vi "HFRR ADV v042.vi"() -> ()   [LabVIEW 2025] (continued)
                n2720 = local read "clk"() -> (w3226:dbl)
                n2721 = Equal?(x=w3226, y=10.0) -> (x = y?=w3228:bool)
                n2722 = case shown="True" w3233 {
                  tunnel: w3232 -> [_ w3359]
                  tunnel: [FALSE ("Boolean 2") TRUE ("Boolean 2")] -> _
                  frame False {
                  }
                  frame True {
                    w3313 = ";" ("Substring")
                    # "Pid out/\nFreq response value"
                    n2723 = local write "act save time"(w3359) -> ()
                    n2724 = local read "FILE"() -> (w3307:string)
                    n2725 = call "file check.vi"("file name in"=w3307) -> ("error out"=w3310:errorcluster, "file name out"=w3305:string)  [unwired: 9 in]
                    n2726 = local read "LVDT STROKE"() -> (w3302:dbl)
                    n2727 = local read "Add up Stroke"() -> (w3300:dbl)
                    n2728 = call "FILE PATH CREATION.vi"("error in"=w3310, "FILE NAME :"=w3305) -> ("FILE OUT"=w3308:path)  [unwired: 8 in, 1 out]
                    n2729 = local read "STROKE Initialize"() -> (w3295:bool)
                    n2730 = Concatenate Strings(w3305, ".dgf" ("Substring")) -> (w3309:string)
                    n2731 = Subtract(x=w3302, y=w3300) -> (x-y=w3301:dbl)
                    n2732 = Absolute Value(x=w3301) -> (abs(x)=w3298:dbl)
                    n2733 = local read "FF 2"() -> (→"Frictional Force ( N )" →"Frictional Force ( N )":dbl)
                    n2734 = Build Path(base path=w3308, name or relative path=w3309) -> (appended path=w3304:path)
                    n2735 = flat-sequence {
                      tunnel: w3298 -> [w3364]
                      tunnel: [w3363] -> w3296
                      tunnel: w3295 -> [w3361]
                      tunnel: [w3366] -> w3297
                      tunnel: w3296 -> [w3366]
                      frame #0 {
                        n2736 = call <vilib>:"Mean PtByPt.vi"("x"=w3364, "sample length"="STROKE FILTER", "initialize"=w3361) -> ("mean"=w3363:dbl)  [unwired: 1 in, 1 out]
                      }
                      frame #1 {
                        "STROKE Initialize" <- FALSE ("STROKE Initialize")
                      }
                    }
                    n2737 = local read "COF 2"() -> (w3318:dbl)
                    "Coefficient of Friction" <- w3318
                    "COF 4" <- w3318
                    "Coefficient of Friction" <- w3318
                    n2738 = local read "TEMP"() -> (w3321:dbl)
                    "Temperature ( Deg C )" <- w3321
                    n2739 = local read "Humidity ( %RH )"() -> (w3320:dbl)
                    n2740 = local read "Frequency ( Hz )"() -> (w3327:dbl)
                    n2741 = local read "LVDT STROKE DISPLAY"() -> (w3299:dbl)
                    n2742 = local read "Elapsed time"() -> (w3352:dbl)
                    n2743 = local read "AIR TEMP"() -> (w3325:dbl)
                    n2744 = local read "PID-out"() -> (w3330:dbl)
                    n2745 = local write "Temperature ( Deg C )"(w3321) -> ()
                    n2746 = Number To Fractional String(number=w3299, width (-)=i16 9 ("precision (6)"), precision (6)=i16 6) -> (F-format string=w3345:string)  [unwired: 1 in]
                    n2747 = Number To Fractional String(number=w3325, width (-)=i16 9 ("precision (6)"), precision (6)=i16 3) -> (F-format string=w3344:string)  [unwired: 1 in]
                    n2748 = Number To Fractional String(number=w3321, width (-)=i16 9 ("precision (6)"), precision (6)=i16 3) -> (F-format string=w3341:string)  [unwired: 1 in]
                    n2749 = Number To Fractional String(number=w3320, width (-)=i16 9 ("precision (6)"), precision (6)=i16 3) -> (F-format string=w3338:string)  [unwired: 1 in]
                    n2750 = Number To Fractional String(number=0.0, width (-)=i16 9 ("precision (6)"), precision (6)=i16 3) -> (F-format string=w3335:string)  [unwired: 1 in]
                    n2751 = Number To Fractional String(number=w3330, width (-)=i16 9 ("precision (6)"), precision (6)=i16 3) -> (F-format string=w3331:string)  [unwired: 1 in]
                    n2752 = Number To Fractional String(number=w3327, width (-)=i16 9 ("precision (6)"), precision (6)=i16 3) -> (F-format string=w3326:string)  [unwired: 1 in]
                    n2753 = Number To Fractional String(number=w3318, width (-)=i16 9 ("precision (6)"), precision (6)=i16 6) -> (F-format string=w3353:string)  [unwired: 1 in]
                    n2754 = Number To Fractional String(number=w3352, width (-)=i16 14 ("precision (6)"), precision (6)=i16 3) -> (F-format string=w3354:string)  [unwired: 1 in]
                    n2755 = Bundle("y"=1.02, "LVDT STROKE DISPLAY"=w3299, "y"=0.98) -> (w3319:T30)  [unwired: 1 in]
                    n2756 = Number To Fractional String(number="Ambient Humidity :", width (-)=i16 9 ("precision (6)"), precision (6)=i16 6) -> (F-format string=w3311:string)  [unwired: 1 in]
                    n2757 = local read "RUN"() -> (w3317:bool)
                    n2758 = case shown="True" w3317 {
                      tunnel: w3319 -> [_ w3370]
                      tunnel: w3299 -> [_ w3369]
                      tunnel: w3299 -> [_ w3367]
                      tunnel: w3299 -> [_ w3368]
                      frame False {
                      }
                      frame True {
                        "Stroke ( mm )" <- w3370
                        "Stroke ( mm )" <- w3370
                        "Stroke 4" <- w3369
                        "Stroke 3" <- w3367
                        "Stroke 2" <- w3368
                        "measured_stroke" <- w3367
                      }
                    }
                    n2759 = Concatenate Strings(w3354, w3313, w3353, w3313, w3345, w3313, w3344, w3313, w3341, w3313, w3338, w3313, w3335, w3313, w3331, w3313, w3326, w3313, w3311, "\r") -> (w3351:string)
                    n2760 = call <vilib>:"Write Characters To File.vi"("append to file? (new file:F)"=TRUE, "character string"=w3351, "file path (dialog if empty)"=w3304) -> ()  [unwired: 2 in, 1 out]
                    "refresh flag" <- TRUE ("refresh flag")
                    "LVDT STROKE Actual" <- w3297
                  }
                }
                n2761 = case shown="True" w3219 {
                  tunnel: w3229 -> [_ w3255]
                  tunnel: w3234 -> [_ w3265]
                  tunnel: [0.0 w3261] -> _
                  tunnel: w3228 -> [_ w3260]
                  tunnel: [0.0 w3259] -> _
                  tunnel: w3218 -> [_ w3259]
                  tunnel: w3232 -> [w3248 _]
                  frame False {
                    n2762 = local write "acq timer"(w3248) -> ()
                    n2763 = local write "Test Duration Status"(0.0 ("Test Duration Status")) -> ()
                  }
                  frame True {
                    n2764 = local read "Set Hz"() -> (w3262:dbl)
                    n2765 = local write "Elapsed time"(w3255) -> ()
                    n2766 = local read "test time"() -> (w3254:dbl)
                    n2767 = Multiply(x=w3265, y=w3262) -> (x*y=w3264:dbl)
                    n2768 = case shown="False" w3260 {
                      tunnel: w3264 -> [w3266 _]
                      tunnel: [w3266 1.0] -> w3261
                      frame False {
                        n2769 = local write "Cycles elapsed"(w3266) -> ()
                      }
                      frame True {
                      }
                    }
                    n2770 = Greater?(x=w3255, y=w3254) -> (0:w3263:bool)
                    n2771 = Subtract(x=w3254, y=w3255) -> (x-y=w3253:dbl)
                    n2772 = Multiply(x=w3253, y=60.0) -> (x*y=w3252:dbl)
                    n2773 = local write "Time Remaining"(w3252) -> ()
                    n2774 = local write "Remaining Time"(w3252) -> ()
                    n2775 = case shown="True" w3263 {
                      frame False {
                      }
                      frame True {
                        n2776 = stacked-sequence {
                          frame #0 {
                            w3271 = T19."Enabled" ("Disabled")
                            w3270 = FALSE ("TEST FILE NAM,E SAVED")
                            w3272 = "" ("FILE")
                            w3273 = TRUE ("Visible")
                            n2777 = local write "Humidity"(FALSE ("Humidity")) -> ()
                            n2778 = local write "RUN"(FALSE ("OK Button 2")) -> ()
                            n2779 = local write "Heater Button"(FALSE ("Heater Button")) -> ()
                            n2780 = local write "Auto Start Test"(FALSE ("Auto Start Test")) -> ()
                            n2781 = local write "TestCompFlg"(TRUE ("StpFlg")) -> ()
                            n2782 = local read "Humidity ( %RH )"() -> (→"Rh After":dbl)
                            n2783 = property on="STOP 2" class="Bool (strict)"("Disabled"=u8 0) -> ()  [unwired: 2 in, 2 out]
                            n2784 = local read "EVENT LOG"() -> (w3278:string)
                            n2785 = call "Event Log.vi"("Content"="Test Completed", "EVENT LOG"=w3278) -> ("EVENT LOG"=w3277:string)  [unwired: 8 in, 1 out]
                            n2786 = property on="RUN" class="Bool (strict)"("Visible"=w3273) -> ()  [unwired: 2 in, 2 out]
                            n2787 = property on="Auto Start Test" class="Bool (strict)"("Visible"=w3273) -> ()  [unwired: 2 in, 2 out]
                            n2788 = local write "Batch Ref Num :"(w3272) -> ()
                            n2789 = local write "FILE"(w3272) -> ()
                            n2790 = local write "EVENT LOG"(w3277) -> ()
                            n2791 = local write "TEST FILE NAM,E SAVED"(w3270) -> ()
                            n2792 = local write "Fuel Discription :"(w3272) -> ()
                            n2793 = local write "START TEMP"(w3270) -> ()
                            n2794 = local write "Remarks :"(w3272) -> ()
                            n2795 = local write "Main Dashboard Buttons"(T1."Imaging" ("Main Dashboard Buttons")) -> ()
                            n2796 = local write "Main Tab"(T2."Adv Scar" ("Main Tab")) -> ()
                            n2797 = property on="FRICVALZ 2" class="Bool (strict)"("DisabledEnum"=w3271) -> ()  [unwired: 2 in, 2 out]
                            n2798 = property on="FRICVALZ 3" class="Bool (strict)"("DisabledEnum"=w3271) -> ()  [unwired: 2 in, 2 out]
                            n2799 = property on="FRICVALZ 4" class="Bool (strict)"("DisabledEnum"=w3271) -> ()  [unwired: 2 in, 2 out]
                          }
                          frame #1 {
                            n2800 = Wait (ms)(milliseconds to wait=u32 1500) -> ()  [unwired: 1 out]
                          }
                          frame #2 {
                            n2801 = local write "Due Write"("VC;0") -> ()
                          }
                          frame #3 {
                            n2802 = Wait (ms)(milliseconds to wait=u32 1500) -> ()  [unwired: 1 out]
                          }
                          frame #4 {
                            n2803 = local write "Due Write"("VC;0") -> ()
                          }
                          frame #5 {
                            n2804 = Wait (ms)(milliseconds to wait=u32 1500) -> ()  [unwired: 1 out]
                          }
                          frame #6 {
                            n2805 = local write "Due Write"("ST;0") -> ()
                          }
                          frame #7 {
                            n2806 = local write "measured_stroke"(0.0 ("measured_stroke")) -> ()
                            n2807 = Wait (ms)(milliseconds to wait=u32 1500) -> ()  [unwired: 1 out]
                          }
                          frame #8 {
                            n2808 = local write "Due Write"("HE;0") -> ()
                            n2809 = local write "Humidity 2"(TRUE ("Humidity")) -> ()
                          }
                        }
                      }
                    }
                    n2810 = Divide(x=w3255, y=w3254) -> (x/y=w3258:dbl)
                    n2811 = Multiply(x=w3258, y=100.0) -> (x*y=w3256:dbl)
                    n2812 = local write "Test Duration Status"(w3256) -> ()
                  }
                }
              }
              frame #2 {
                n2813 = case shown="True" "Heater Button" {
                  tunnel: [0.0 ("output") w3393] -> w3371
                  frame False {
                    w3374 = TRUE ("tmpchk")
                    n2814 = local read "TEMP"() -> (w3375:dbl)
                    n2815 = local write "Temp ini"(w3375) -> ()
                    n2816 = local write "Reset 4"(w3374) -> ()
                    n2817 = local write "tmpchk"(w3374) -> ()
                    n2818 = local write "reinit"(TRUE ("reinit")) -> ()
                    n2819 = local write "manual temp log"(TRUE ("manual temp log")) -> ()
                  }
                  frame True {
                    # "Logic to turn off\nthe heater when \ntemp is not rising.\nTime - 60 sec\nDelta t- 5°c"
                    n2820 = local read "Temp ini"() -> (w3382:dbl)
                    n2821 = local read "Auto Start Test"() -> (w3378:bool)
                    n2822 = Less?(x=w3382, y=53.0) -> (x < y?=w3380:bool)
                    n2823 = case shown="False" w3378 {
                      frame False {
                        n2824 = local read "Set Temp"() -> (w3402:dbl)
                        n2825 = local read "TEMP"() -> (w3401:dbl)
                        n2826 = Subtract(x=w3402, y=w3401) -> (x-y=w3400:dbl)
                        n2827 = Absolute Value(x=w3400) -> (abs(x)=w3399:dbl)
                        n2828 = Less?(x=w3399, y=0.5) -> (x < y?=w3397:bool)
                        n2829 = case shown="True" w3397 {
                          tunnel: "manual temp log" -> [_ w3403]
                          frame False {
                          }
                          frame True {
                            n2830 = case shown="True" w3403 {
                              selector: w3403 -> [_ w3404]
                              frame False {
                              }
                              frame True {
                                # "#Event log"
                                n2831 = Not(x=w3404) -> (.not. x?=w3405:bool)
                                n2832 = local write "manual temp log"(w3405) -> ()
                                n2833 = local read "EVENT LOG"() -> (w3408:string)
                                n2834 = call "Event Log.vi"("Content"="Target Temperature reached", "EVENT LOG"=w3408) -> ("EVENT LOG"=w3407:string)  [unwired: 8 in, 1 out]
                                n2835 = local write "EVENT LOG"(w3407) -> ()
                              }
                            }
                          }
                        }
                      }
                      frame True {
                        n2836 = local write "manual temp log"(TRUE ("manual temp log")) -> ()
                      }
                    }
                    n2837 = And(x="tmpchk", y=w3380) -> (x .and. y?=w3383:bool)
                    n2838 = case shown="True" w3383 {
                      frame False {
                      }
                      frame True {
                        n2839 = call "Elapsed Time8"("Time Target (s)"=300.0, "Reset"="Reset 4") -> ("Time has Elapsed"=w3410:bool)  [unwired: 10 in, 7 out]
                        n2840 = flat-sequence {
                          tunnel: w3410 -> [_]
                          frame #0 {
                            n2841 = local write "Reset 4"(FALSE ("Reset 4")) -> ()
                          }
                        }
                        n2842 = case shown="True" w3410 {
                          frame False {
                          }
                          frame True {
                            n2843 = local read "Temp ini"() -> (w3417:dbl)
                            n2844 = Add(x=w3417, y=5.0) -> (x+y=w3415:dbl)
                            n2845 = local read "TEMP"() -> (w3418:dbl)
                            n2846 = Greater?(x=w3418, y=w3415) -> (0:w3416:bool)
                            n2847 = case shown="False" w3416 {
                              frame False {
                                n2848 = local write "Heater Button"(FALSE ("Heater Button")) -> ()
                              }
                              frame True {
                                n2849 = local write "tmpchk"(FALSE ("tmpchk")) -> ()
                              }
                            }
                          }
                        }
                      }
                    }
                    n2850 = local read "Set Temp"() -> (w3391:dbl)
                    n2851 = local read "TEMP"() -> (w3385:dbl)
                    n2852 = call-poly <vilib>:"PID.vi"("reinitialize? (F)"="reinit", "dt (s)"=-1.0, "process variable"=w3385, "setpoint"=w3391) -> ("output"=w3388:dbl)  [unwired: 6 in, 1 out]
                    n2853 = Subtract(x=w3391, y=w3385) -> (x-y=w3392:dbl)
                    n2854 = Add(x=w3391, y=0.5) -> (x+y=w3389:dbl)
                    n2855 = Greater Or Equal?(x=w3385, y=w3389) -> ()  [unwired: 1 out]
                    n2856 = Select(t=0.0, s=FALSE, f=w3388) -> (s? t:f=w3387:dbl)
                    "PID output" <- w3387
                    n2857 = flat-sequence {
                      tunnel: w3387 -> [w3421]
                      tunnel: [w3421] -> w3393
                      frame #0 {
                        n2858 = local write "reinit"(FALSE ("reinit")) -> ()
                      }
                    }
                    n2859 = Bundle(w3392, "output"=w3387, "TEMP"=w3385) -> ()  [unwired: 1 in, 1 out]
                  }
                }
                "PID-out" <- w3371
              }
              frame #3 {
                n2860 = local read "TEMP"() -> (w3423:dbl)
                n2861 = Greater Or Equal?(x=w3423, y="Set Temp 2") -> (x >= y?=w3428:bool)
                n2862 = case shown="True" w3428 {
                  tunnel: [FALSE TRUE] -> w3426
                  frame False {
                  }
                  frame True {
                  }
                }
                "Status 13" <- w3426
                n2863 = And(x=w3426, y="trip1 8") -> (x .and. y?=w3425:bool)
                n2864 = case shown="True" w3425 {
                  frame False {
                    n2865 = local write "Heater Trip Temp"(TRUE ("Heater Trip Temp")) -> ()
                  }
                  frame True {
                    w3431 = FALSE ("OK Button 2")
                    n2866 = case shown="True" "Heater Trip Temp" {
                      selector: "Heater Trip Temp" -> [_ w3433]
                      frame False {
                      }
                      frame True {
                        n2867 = Not(x=w3433) -> (.not. x?=w3432:bool)
                        n2868 = local read "EVENT LOG"() -> (w3436:string)
                        n2869 = local write "Heater Trip Temp"(w3432) -> ()
                        n2870 = call "Event Log.vi"("Content"="Heater Trip", "EVENT LOG"=w3436) -> ("EVENT LOG"=w3435:string)  [unwired: 8 in, 1 out]
                        n2871 = local write "EVENT LOG"(w3435) -> ()
                      }
                    }
                    n2872 = local write "RUN"(w3431) -> ()
                    n2873 = property on="Auto Start Test" class="Bool (strict)"("Value"=w3431) -> ()  [unwired: 2 in, 2 out]
                    n2874 = local write "Heater Button"(w3431) -> ()
                  }
                }
              }
            }
            n2875 = case shown="False" w3142 {
              frame False {
                n2876 = disable-structure shown="Disabled" {
                  frame Disabled {
                    n2877 = stacked-sequence {
                      frame #0 {
                        n2878 = local write "RUN"(FALSE ("OK Button 2")) -> ()
                      }
                      frame #1 {
                      }
                    }
                  }
                  frame Enabled {
                  }
                }
              }
              frame True {
              }
            }
          }
        }
        n2879 = local read "Reset Graph"() -> (w3039:bool)
        n2880 = case shown="True" w3039 {
          selector: w3039 -> [_ w3056]
          frame False {
          }
          frame True {
            w3070 = 0.0 ("X Scale.Range:Maximum")
            n2881 = Not(x=w3056) -> (.not. x?=w3055:bool)
            n2882 = local write "Reset Graph"(w3055) -> ()
            n2883 = property on="Electrical Contact Resistance ( % )" class="WFChart (strict)"("XScale.Maximum"=600.0 ("X Scale.Range:Maximum"), "XScale.Minimum"=0.0 ("X Scale.Range:Minimum"), "YScale.Maximum"=100.0 ("Y Scale.Range:Maximum"), "YScale.Minimum"=0.0 ("Y Scale.Range:Minimum")) -> ()  [unwired: 2 in, 2 out]
            n2884 = property on="Frictional Force ( N )" class="WFChart (strict)"("XScale.Maximum"=600.0 ("X Scale.Range:Maximum"), "XScale.Minimum"=0.0 ("X Scale.Range:Minimum"), "YScale.Maximum"=100.0 ("Y Scale.Range:Maximum"), "YScale.Minimum"=0.0 ("Y Scale.Range:Minimum")) -> ()  [unwired: 2 in, 2 out]
            n2885 = property on="Temperature ( Deg C )" class="WFChart (strict)"("XScale.Maximum"=600.0 ("X Scale.Range:Maximum"), "XScale.Minimum"=0.0 ("X Scale.Range:Minimum"), "YScale.Maximum"=100.0 ("Y Scale.Range:Maximum"), "YScale.Minimum"=0.0 ("Y Scale.Range:Minimum")) -> ()  [unwired: 2 in, 2 out]
            n2886 = property on="Stroke ( mm )" class="WFChart (strict)"("XScale.Maximum"=600.0 ("X Scale.Range:Maximum"), "XScale.Minimum"=0.0 ("X Scale.Range:Minimum"), "YScale.Maximum"=100.0 ("Y Scale.Range:Maximum"), "YScale.Minimum"=0.0 ("Y Scale.Range:Minimum")) -> ()  [unwired: 2 in, 2 out]
            n2887 = property on="Coefficient of Friction" class="WFChart (strict)"("XScale.Maximum"=600.0 ("X Scale.Range:Maximum"), "XScale.Minimum"=0.0 ("X Scale.Range:Minimum"), "YScale.Maximum"=100.0 ("Y Scale.Range:Maximum"), "YScale.Minimum"=0.0 ("Y Scale.Range:Minimum")) -> ()  [unwired: 2 in, 2 out]
            n2888 = property on="Electrical Contact Resistance ( % )" class="WFChart (strict)"("XScale.Minimum"=0.0 ("X Scale.Range:Minimum"), "XScale.Maximum"=600.0 ("X Scale.Range:Maximum"), "YScale.Minimum"=0.0 ("Y Scale.Range:Minimum"), "YScale.Maximum"=100.0 ("Y Scale.Range:Maximum")) -> ()  [unwired: 2 in, 2 out]
            n2889 = property on="Temperature ( Deg C )" class="WFChart (strict)"("XScale.Minimum"=0.0 ("X Scale.Range:Minimum"), "XScale.Maximum"=600.0 ("X Scale.Range:Maximum"), "YScale.Minimum"=0.0 ("Y Scale.Range:Minimum"), "YScale.Maximum"=100.0 ("Y Scale.Range:Maximum")) -> ()  [unwired: 2 in, 2 out]
            n2890 = property on="Coefficient of Friction" class="WFChart (strict)"("XScale.Minimum"=0.0 ("X Scale.Range:Minimum"), "XScale.Maximum"=600.0 ("X Scale.Range:Maximum"), "YScale.Maximum"=1.0 ("X Scale.Range:Minimum"), "YScale.Minimum"=0.0 ("X Scale.Range:Minimum")) -> ()  [unwired: 2 in, 2 out]
            n2891 = property on="Frictional Force ( N )" class="WFChart (strict)"("XScale.Maximum"=600.0 ("X Scale.Range:Maximum"), "XScale.Minimum"=w3070, "YScale.Maximum"=10.0 ("Y Scale.Range:Maximum"), "YScale.Minimum"=w3070) -> ()  [unwired: 2 in, 2 out]
            n2892 = property on="Stroke ( mm )" class="WFChart (strict)"("XScale.Maximum"=600.0 ("X Scale.Range:Maximum"), "XScale.Minimum"=0.0 ("X Scale.Range:Minimum"), "YScale.Maximum"=100.0 ("Y Scale.Range:Maximum"), "YScale.Minimum"=0.0 ("Y Scale.Range:Minimum")) -> ()  [unwired: 2 in, 2 out]
          }
        }
      }
      frame "Compare Files" {
        # "Elapsed time\ncof\nstroke\nAir temp\nTemp\nHumidity"
        n2893 = case shown="True" "RSTV1 2" {
          frame False {
          }
          frame True {
            n2894 = property on="Humidity ( %RH )" class="XYGraph (strict)"("Y Scale.Display Format:Precision"=u8 0 ("Y Scale.Format & Precision:Precision")) -> ()  [unwired: 2 in, 2 out]
            n2895 = property on="Humidity ( %RH )" class="XYGraph (strict)"("X Scale.Range:Minimum"=0.0, "X Scale.Range:Maximum"=75.0, "Y Scale.Range:Minimum"=48.0, "Y Scale.Range:Maximum"=58.0) -> ()  [unwired: 2 in, 2 out]
          }
        }
        n2896 = case shown="True" "RST CP 2" {
          frame False {
          }
          frame True {
            n2897 = property on="XY Graph 13" class="XYGraph (strict)"("Y Scale.Display Format:Precision"=u8 0 ("Y Scale.Format & Precision:Precision")) -> ()  [unwired: 2 in, 2 out]
            n2898 = property on="XY Graph 13" class="XYGraph (strict)"("X Scale.Range:Minimum"=0.0, "X Scale.Range:Maximum"=75.0, "Y Scale.Range:Minimum"=0.0, "Y Scale.Range:Maximum"=100.0) -> ()  [unwired: 2 in, 2 out]
          }
        }
        n2899 = case shown="True" "RST CP" {
          frame False {
          }
          frame True {
            n2900 = property on="Sample Temperature ( °C )" class="XYGraph (strict)"("Y Scale.Display Format:Precision"=u8 2 ("Y Scale.Format & Precision:Precision")) -> ()  [unwired: 2 in, 2 out]
            n2901 = property on="Sample Temperature ( °C )" class="XYGraph (strict)"("X Scale.Range:Minimum"=0.0, "X Scale.Range:Maximum"=75.0, "Y Scale.Range:Minimum"=58.0, "Y Scale.Range:Maximum"=62.0) -> ()  [unwired: 2 in, 2 out]
          }
        }
        n2902 = case shown="True" "RSTV1 3" {
          frame False {
          }
          frame True {
            n2903 = property on="Air Temperature  ( °C )" class="XYGraph (strict)"("Y Scale.Display Format:Precision"=u8 2 ("Y Scale.Format & Precision:Precision")) -> ()  [unwired: 2 in, 2 out]
            n2904 = property on="Air Temperature  ( °C )" class="XYGraph (strict)"("X Scale.Range:Minimum"=0.0 ("Y Scale.Range:Minimum"), "X Scale.Range:Maximum"=75.0 ("Y Scale.Range:Maximum"), "Y Scale.Range:Minimum"=20.0 ("X Scale.Range:Minimum"), "Y Scale.Range:Maximum"=26.0 ("X Scale.Range:Maximum")) -> ()  [unwired: 2 in, 2 out]
          }
        }
        n2905 = case shown="True" "RSTV1 4" {
          frame False {
          }
          frame True {
            n2906 = property on="Stroke ( mm )" class="XYGraph (strict)"("Y Scale.Display Format:Precision"=u8 2 ("Y Scale.Format & Precision:Precision")) -> ()  [unwired: 2 in, 2 out]
            n2907 = property on="Stroke ( mm )" class="XYGraph (strict)"("X Scale.Range:Minimum"=0.0 ("Y Scale.Range:Maximum"), "X Scale.Range:Maximum"=75.0 ("X Scale.Range:Minimum"), "Y Scale.Range:Minimum"=0.98, "Y Scale.Range:Maximum"=1.02) -> ()  [unwired: 2 in, 2 out]
          }
        }
        n2908 = case shown="True" "rstv2" {
          frame False {
          }
          frame True {
            n2909 = property on="Coefficient Of Friction" class="XYGraph (strict)"("Y Scale.Display Format:Precision"=u8 3 ("Y Scale.Format & Precision:Precision")) -> ()  [unwired: 2 in, 2 out]
            n2910 = property on="Coefficient Of Friction" class="XYGraph (strict)"("X Scale.Range:Minimum"=0.0 ("Y Scale.Range:Maximum"), "X Scale.Range:Maximum"=75.0, "Y Scale.Range:Minimum"=0.0, "Y Scale.Range:Maximum"=1.0 ("X Scale.Range:Minimum")) -> ()  [unwired: 2 in, 2 out]
          }
        }
        n2911 = case shown="True" "RST CP 3" {
          frame False {
          }
          frame True {
            n2912 = property on="Air Temp ( °C ) vs Humidity ( % RH )" class="XYGraph (strict)"("X Scale.Range:Minimum"=18.0, "X Scale.Range:Maximum"=28.0 ("X Scale.Range:Minimum"), "Y Scale.Range:Minimum"=30.0 ("X Scale.Range:Minimum"), "Y Scale.Range:Maximum"=70.0 ("X Scale.Range:Minimum")) -> ()  [unwired: 2 in, 2 out]
          }
        }
        n2913 = case shown="True" "OPEN 1" {
          frame False {
          }
          frame True {
            (unwired) 0  # existing file
            w3712 = "Choose a datalog file to open"  # prompt
            n2914 = local write "OPEN 1"(FALSE ("OPEN 1")) -> ()
            n2915 = String To Path(string="C:\\LAB-IQ\\Data\\") -> (path=w3697:path)
            n2916 = File Dialog(6:"*.dgf" ("pattern"), 7:w3712, 11:w3697) -> (0:w3695:errorcluster, 3:w3703:path)  [unwired: 4 in, 2 out]
            n2917 = Unbundle(w3695) -> ()  [unwired: 3 out]
            n2918 = Strip Path(path=w3703) -> (name=w3702:string)  [unwired: 1 out]
            n2919 = Path To String(path=w3703) -> (string=w3698:string)
            "string1" <- w3698
            n2920 = Match Pattern(string=w3702, regular expression=".dgf") -> (before substring=→"String Control":string)  [unwired: 1 in, 3 out]
            n2921 = Match Pattern(string=w3698, regular expression=".dgf" ("substring (\"\")")) -> (before substring=w3708:string)  [unwired: 1 in, 3 out]
            n2922 = Concatenate Strings(w3708, ".duf" ("Substring")) -> (w3704:string)
            n2923 = String To Path(string=w3704) -> (path=w3709:path)
            n2924 = call <vilib>:"Read Characters From File.vi"("file path (dialog if empty)"=w3709, "start of read offset (chars.:0)"=60 ("start of read offset (chars.: 0)")) -> ("character string"=→"String Control 2":string)  [unwired: 4 in, 3 out]
          }
        }
        n2925 = case shown="True" "OPEN 2" {
          frame False {
          }
          frame True {
            (unwired) 0  # existing file
            w3730 = "Choose a datalog file to open"  # prompt
            n2926 = local write "OPEN 2"(FALSE ("OPEN 1")) -> ()
            n2927 = String To Path(string="C:\\LAB-IQ\\Data\\") -> (path=w3715:path)
            n2928 = File Dialog(6:"*.dgf" ("pattern"), 7:w3730, 11:w3715) -> (0:w3713:errorcluster, 3:w3721:path)  [unwired: 4 in, 2 out]
            n2929 = Unbundle(w3713) -> ()  [unwired: 3 out]
            n2930 = Strip Path(path=w3721) -> (name=w3719:string)  [unwired: 1 out]
            n2931 = Path To String(path=w3721) -> (string=w3716:string)
            "string1 2" <- w3716
            n2932 = Match Pattern(string=w3719, regular expression=".dgf") -> (before substring=→"String Control 3":string)  [unwired: 1 in, 3 out]
            n2933 = Match Pattern(string=w3716, regular expression=".dgf" ("substring (\"\")")) -> (before substring=w3727:string)  [unwired: 1 in, 3 out]
            n2934 = Concatenate Strings(w3727, ".duf" ("Substring")) -> (w3724:string)
            n2935 = String To Path(string=w3724) -> (path=w3722:path)
            n2936 = call <vilib>:"Read Characters From File.vi"("file path (dialog if empty)"=w3722, "start of read offset (chars.:0)"=60 ("start of read offset (chars.: 0)")) -> ("character string"=→"String Control 4":string)  [unwired: 4 in, 3 out]
          }
        }
        n2937 = case shown="True" "OPEN 3" {
          frame False {
          }
          frame True {
            (unwired) 0  # existing file
            w3748 = "Choose a datalog file to open"  # prompt
            n2938 = local write "OPEN 3"(FALSE ("OPEN 1")) -> ()
            n2939 = String To Path(string="C:\\LAB-IQ\\Data\\") -> (path=w3733:path)
            n2940 = File Dialog(6:"*.dgf" ("pattern"), 7:w3748, 11:w3733) -> (0:w3731:errorcluster, 3:w3739:path)  [unwired: 4 in, 2 out]
            n2941 = Unbundle(w3731) -> ()  [unwired: 3 out]
            n2942 = Strip Path(path=w3739) -> (name=w3737:string)  [unwired: 1 out]
            n2943 = Path To String(path=w3739) -> (string=w3734:string)
            "string1 3" <- w3734
            n2944 = Match Pattern(string=w3737, regular expression=".dgf") -> (before substring=→"String Control 5":string)  [unwired: 1 in, 3 out]
            n2945 = Match Pattern(string=w3734, regular expression=".dgf" ("substring (\"\")")) -> (before substring=w3744:string)  [unwired: 1 in, 3 out]
            n2946 = Concatenate Strings(w3744, ".duf" ("Substring")) -> (w3741:string)
            n2947 = String To Path(string=w3741) -> (path=w3745:path)
            n2948 = call <vilib>:"Read Characters From File.vi"("file path (dialog if empty)"=w3745, "start of read offset (chars.:0)"=60 ("start of read offset (chars.: 0)")) -> ("character string"=→"String Control 6":string)  [unwired: 4 in, 3 out]
          }
        }
        n2949 = case shown="True" "OPEN 4" {
          frame False {
          }
          frame True {
            (unwired) 0  # existing file
            w3766 = "Choose a datalog file to open"  # prompt
            n2950 = local write "OPEN 4"(FALSE ("OPEN 1")) -> ()
            n2951 = String To Path(string="C:\\LAB-IQ\\Data\\") -> (path=w3751:path)
            n2952 = File Dialog(6:"*.dgf" ("pattern"), 7:w3766, 11:w3751) -> (0:w3749:errorcluster, 3:w3757:path)  [unwired: 4 in, 2 out]
            n2953 = Unbundle(w3749) -> ()  [unwired: 3 out]
            n2954 = Strip Path(path=w3757) -> (name=w3755:string)  [unwired: 1 out]
            n2955 = Path To String(path=w3757) -> (string=w3752:string)
            "string1 4" <- w3752
            n2956 = Match Pattern(string=w3755, regular expression=".dgf") -> (before substring=→"String Control 7":string)  [unwired: 1 in, 3 out]
            n2957 = Match Pattern(string=w3752, regular expression=".dgf" ("substring (\"\")")) -> (before substring=w3762:string)  [unwired: 1 in, 3 out]
            n2958 = Concatenate Strings(w3762, ".duf" ("Substring")) -> (w3759:string)
            n2959 = String To Path(string=w3759) -> (path=w3763:path)
            n2960 = call <vilib>:"Read Characters From File.vi"("file path (dialog if empty)"=w3763, "start of read offset (chars.:0)"=60 ("start of read offset (chars.: 0)")) -> ("character string"=→"String Control 8":string)  [unwired: 4 in, 3 out]
          }
        }
      }
      frame "About" {
        # "Elapsed time\ncof\nstroke\nmean pos\nTemp\nHumidity"
        n2961 = disable-structure shown="Disabled" {
          frame Disabled {
            n2962 = case shown="True" "Export" {
              frame False {
              }
              frame True {
                w3788 = "                                      " ("string")
                w3790 = "\r"
                (unwired) i16 6 ("width (-)")
                w3867 = "\r"
                w3799 = "\r"
                n2963 = local write "Export"(FALSE ("Export")) -> ()
                n2964 = local read "String 29"() -> (w3836:string)
                n2965 = local read "String 34"() -> (w3824:string)
                n2966 = local read "String 35"() -> (w3819:string)
                n2967 = local read "String 37"() -> (w3815:string)
                n2968 = local read "String 36"() -> (w3812:string)
                n2969 = local read "String 38"() -> (w3809:string)
                n2970 = local read "String 39"() -> (w3806:string)
                n2971 = Match Pattern(string=w3836, regular expression=".dwm") -> (before substring=w3832:string)  [unwired: 1 in, 3 out]
                "before substring" <- w3832
                n2972 = local read "S 38"() -> (w3827:string)
                n2973 = local read "S 39"() -> (w3820:string)
                n2974 = local read "Temperature before test 2"() -> (w3856:dbl)
                n2975 = local read "Temperature after test 2"() -> (w3861:dbl)
                n2976 = local read "Humidity before test 2"() -> (w3842:dbl)
                n2977 = local read "Humidity after test 2"() -> (w3857:dbl)
                n2978 = local read "MWSD 2"() -> (w3853:dbl)
                n2979 = local read "WS1.4 2"() -> (w3869:dbl)
                n2980 = local read "HCF 2"() -> (w3865:dbl)
                n2981 = local read "AVP 2"() -> (w3854:dbl)
                n2982 = Concatenate Strings("1," ("string"), w3827) -> (w3826:string)
                n2983 = Concatenate Strings("2," ("string"), w3824) -> (w3823:string)
                n2984 = Concatenate Strings("3," ("string"), w3820) -> (w3822:string)
                n2985 = Concatenate Strings("4," ("string"), w3819) -> (w3818:string)
                n2986 = Concatenate Strings("5," ("string"), w3815) -> (w3816:string)
                n2987 = Concatenate Strings("6," ("string"), w3812) -> (w3813:string)
                n2988 = Concatenate Strings("7," ("string"), w3809) -> (w3810:string)
                n2989 = Concatenate Strings("8," ("string"), w3806) -> (w3807:string)
                n2990 = local read "Sample ID"() -> (w3874:string)
                n2991 = case shown="\"xlx\"" "Select File Type" {
                  tunnel: w3832 -> [w3877 w3879 w3881]
                  tunnel: [w3875 w3880 w3882] -> w3831
                  frame "xlx" {
                    n2992 = Concatenate Strings(w3877, ".xls" ("string")) -> (w3875:string)
                  }
                  frame "csv" {
                    n2993 = Concatenate Strings(w3879, ".csv" ("string")) -> (w3880:string)
                  }
                  frame "txt" {
                    n2994 = Concatenate Strings(w3881, ".txt" ("string")) -> (w3882:string)
                  }
                }
                n2995 = local read "Test Date"() -> (w3873:string)
                n2996 = local read "String 45"() -> (w3787:string)
                n2997 = local read "String 31"() -> (w3872:string)
                n2998 = local read "String 32"() -> (w3871:string)
                n2999 = local read "TITTLE"() -> (w3795:string)
                n3000 = Number To Fractional String(number=w3842, width (-)=i16 6, precision (6)=i16 2) -> (F-format string=w3841:string)  [unwired: 1 in]
                n3001 = Number To Fractional String(number=w3856, width (-)=i16 6, precision (6)=i16 2) -> (F-format string=w3862:string)  [unwired: 1 in]
                n3002 = Number To Fractional String(number=w3857, width (-)=i16 6, precision (6)=i16 2) -> (F-format string=w3855:string)  [unwired: 1 in]
                n3003 = Number To Fractional String(number=w3861, width (-)=i16 6, precision (6)=i16 2) -> (F-format string=w3860:string)  [unwired: 1 in]
                n3004 = Number To Fractional String(number=w3853, width (-)=i16 6, precision (6)=i16 2) -> (F-format string=w3851:string)  [unwired: 1 in]
                n3005 = Number To Fractional String(number=w3854, width (-)=i16 6, precision (6)=i16 2) -> (F-format string=w3852:string)  [unwired: 1 in]
                n3006 = Number To Fractional String(number=w3865, width (-)=i16 6, precision (6)=i16 2) -> (F-format string=w3866:string)  [unwired: 1 in]
                n3007 = Number To Fractional String(number=w3869, precision (6)=i16 2) -> (F-format string=w3870:string)  [unwired: 2 in]
                n3008 = local read "s.NO"() -> (w3789:string)
                n3009 = Concatenate Strings("=" ("string"), w3795) -> (w3794:string)
                n3010 = Concatenate Strings("S.No," ("string"), "                                       Parameters" ("string")) -> (w3800:string)
                n3011 = Concatenate Strings(w3867, w3826, w3841, w3867, w3823, w3862, w3867, w3822, w3855, w3867, w3818, w3860, w3867, w3816, w3851, w3867, w3813, w3852, w3867, w3810, w3866, w3867, w3807, w3870) -> (w3829:string)
                n3012 = Concatenate Strings(w3799, "," ("string"), w3787, w3789, w3788, w3871, w3874, w3788, w3872, w3873, w3799) -> (w3797:string)
                n3013 = local read "Tested by"() -> (w3803:string)
                n3014 = local read "String 33"() -> (w3804:string)
                n3015 = Concatenate Strings("," ("string"), "                                                                             " ("string")) -> (w3792:string)
                n3016 = Concatenate Strings(w3794, w3790, w3797, w3790, w3800, w3829, w3790, w3792, w3804, w3803) -> (→"export":string)
                n3017 = String To Path(string=w3831) -> (path=w3838:path)
                n3018 = local read "export"() -> (w3833:string)
                n3019 = call <vilib>:"Write Characters To File.vi"("append to file? (new file:F)"=FALSE, "character string"=w3833, "file path (dialog if empty)"=w3838) -> ()  [unwired: 2 in, 1 out]
              }
            }
          }
          frame Enabled {
          }
        }
        n3020 = case shown="True" "OK Button 17" {
          frame False {
          }
          frame True {
            (unwired) 0  # existing file
            w4091 = "Choose a datalog file to open"  # prompt
            n3021 = local write "OK Button 17"(FALSE ("OK Button 17")) -> ()
            n3022 = local read "String"() -> (w4086:string)
            n3023 = String To Path(string=w4086) -> (path=w4087:path)
            n3024 = File Dialog(6:"*.duf" ("pattern"), 7:w4091, 11:w4087) -> (0:w4078:errorcluster, 3:w4097:path)  [unwired: 4 in, 2 out]
            n3025 = Unbundle(w4078) -> ()  [unwired: 3 out]
            n3026 = Open/Create/Replace File "Open File"(file path (use dialog)=w4097) -> (refnum out=w4089:refnum<file>)  [unwired: 5 in, 2 out]
            n3027 = Strip Path(path=w4097) -> (name=w4095:string)  [unwired: 1 out]
            n3028 = Path To String(path=w4097) -> (string=w4080:string)
            n3029 = while {
              tunnel: w4089 -> [w4101]
              i -> [w4098]
              stop <- w4099 continue-if-true
              (unwired) TRUE ("line mode (F)")
              n3030 = Read from Text File "Read File"(file (use dialog)=w4101) -> (text=w4100:string)  [unwired: 3 in, 3 out]
              n3031 = local write "Numeric 16"(w4098) -> ()
              n3032 = String Length(string=w4100) -> (length=w4103:i32)
              n3033 = Greater?(x=w4103, y=1) -> (0:w4099:bool)
            }
            n3034 = local write "String 29"(w4080) -> ()
            n3035 = Search and Replace String(input string=w4080, search string=".duf", replace string=".dgf" ("replace string (\"\")")) -> (result string=→"String Indicator 4":string)  [unwired: 5 in, 3 out]
            n3036 = Match Pattern(string=w4095, regular expression=".dwm") -> (before substring=w4079:string)  [unwired: 1 in, 3 out]
            "String Indicator" <- w4079
            n3037 = Match Pattern(string=w4080, regular expression=".dwm" ("substring (\"\")")) -> (before substring=w4081:string)  [unwired: 1 in, 3 out]
            "String Indicator 3" <- w4081
            n3038 = local write "TITTLE 2"(w4079) -> ()
            n3039 = String To Path(string=w4081) -> (path=w4088:path)
            "path" <- w4088
            n3040 = call <vilib>:"Read Characters From File.vi"("file path (dialog if empty)"=w4088, "start of read offset (chars.:0)"=60 ("start of read offset (chars.: 0)")) -> ("character string"=→"String Indicator 2":string)  [unwired: 4 in, 3 out]
          }
        }
        n3041 = call <vilib>:"Query Available Printers.vi"() -> ("system configured printers"=w3780:string[])  [unwired: 9 in, 2 out]
        "System Configured Printers 2" <- w3780
        n3042 = local read "OK Button 16"() -> (w3777:bool)
        n3043 = case shown="True" "OK Button 16" {
          frame False {
          }
          frame True {
            n3044 = stacked-sequence {
              frame #0 {
                n3045 = local read "Numeric 16"() -> (w4105:i32)
                n3046 = local write "Numeric 10"(w4105) -> ()
              }
              frame #1 {
                n3047 = local read "String 29"() -> (w4108:string)
                n3048 = String To Path(string=w4108) -> (path=w4107:path)
                n3049 = Open/Create/Replace File "Open File"(file path (use dialog)=w4107) -> (refnum out=w4109:refnum<file>)  [unwired: 5 in, 2 out]
                n3050 = for {
                  N: 16 -> [_]
                  tunnel: w4109 -> [w4116]
                  i -> [w4112]
                  (unwired) TRUE ("line mode (F)")
                  n3051 = Read from Text File "Read File"(file (use dialog)=w4116) -> (text=w4110:string)  [unwired: 3 in, 3 out]
                  n3052 = Match Pattern(string=w4110, regular expression="(") -> (after substring=w4115:string)  [unwired: 1 in, 3 out]
                  n3053 = Match Pattern(string=w4115, regular expression=")") -> (before substring=w4111:string)  [unwired: 1 in, 3 out]
                  n3054 = case shown="1" w4112 {
                    tunnel: w4111 -> [w4117 w4118 _ _ w4119 w4120 w4121 w4123 w4125 w4127 w4129 w4131 w4133 w4135 _]
                    tunnel: w4110 -> [_ _ _ _ _ _ _ _ _ _ _ _ _ _ _]
                    frame 0 {
                      "TITTLE" <- w4117
                    }
                    frame 1 {
                      "Sample ID" <- w4118
                    }
                    frame 2 {
                    }
                    frame 3 {
                    }
                    frame 4 {
                      "Test Date" <- w4119
                    }
                    frame 5 {
                      "Tested by" <- w4120
                    }
                    frame 6 {
                      n3055 = Fract/Exp String To Number(string=w4121) -> (number=→"Humidity before test 2":dbl)  [unwired: 3 in, 1 out]
                    }
                    frame 7 {
                      n3056 = Fract/Exp String To Number(string=w4123) -> (number=→"Temperature before test 2":dbl)  [unwired: 3 in, 1 out]
                    }
                    frame 8 {
                      n3057 = Fract/Exp String To Number(string=w4125) -> (number=→"Humidity after test 2":dbl)  [unwired: 3 in, 1 out]
                    }
                    frame 9 {
                      n3058 = Fract/Exp String To Number(string=w4127) -> (number=→"Temperature after test 2":dbl)  [unwired: 3 in, 1 out]
                    }
                    frame 10 {
                      n3059 = Fract/Exp String To Number(string=w4129) -> (number=→"MWSD 2":dbl)  [unwired: 3 in, 1 out]
                    }
                    frame 11 {
                      n3060 = Fract/Exp String To Number(string=w4131) -> (number=→"AVP 2":dbl)  [unwired: 3 in, 1 out]
                    }
                    frame 12 {
                      n3061 = Fract/Exp String To Number(string=w4133) -> (number=→"HCF 2":dbl)  [unwired: 3 in, 1 out]
                    }
                    frame 13 {
                      n3062 = Fract/Exp String To Number(string=w4135) -> (number=→"WS1.4 2":dbl)  [unwired: 3 in, 1 out]
                    }
                    frame 14, Default {
                    }
                  }
                }
              }
              frame #2 {
              }
            }
            n3063 = local write "OK Button 16"(FALSE ("OK Button 13")) -> ()
          }
        }
        n3064 = Index Array(array=w3780, index="Select Printer 3") -> (element=w3782:string)
        "Selected Printer" <- w3782
        n3065 = case shown="True" w3777 {
          frame False {
          }
          frame True {
            n3066 = flat-sequence {
              frame #0 {
              }
              frame #1 {
                n3067 = Wait (ms)(milliseconds to wait=u32 100) -> ()  [unwired: 1 out]
              }
              frame #2 {
                n3068 = local write "OK Button 16"(FALSE ("Print 3")) -> ()
              }
            }
          }
        }
        n3069 = case shown="True" "Print" {
          tunnel: w3782 -> [_ w4074]
          frame False {
          }
          frame True {
            (unwired) i16 6 ("width (-)")
            (unwired) "TESTED BY : "
            (unwired) "TESTED DATE :"
            (unwired) "SAMPLE ID : "
            (unwired) "SAMPLE DESIGN : "
            w4032 = "\r"
            w4049 = "\r"
            # "add image"
            n3070 = local read "Sample ID"() -> (w4022:string)
            n3071 = local read "Tested by"() -> (w4025:string)
            n3072 = local read "String 34"() -> (w4012:string)
            n3073 = local read "String 45"() -> (w3992:string)
            n3074 = local read "String 35"() -> (w4007:string)
            n3075 = local read "String 37"() -> (w4005:string)
            n3076 = local read "String 32"() -> (w4027:string)
            n3077 = local read "String 36"() -> (w4002:string)
            n3078 = local read "String 31"() -> (w4026:string)
            n3079 = local read "Test Date"() -> (w4023:string)
            n3080 = local read "String 33"() -> (w4028:string)
            n3081 = local read "String 38"() -> (w3998:string)
            n3082 = local read "String 39"() -> (w3995:string)
            n3083 = local write "Print"(FALSE ("Print FF")) -> ()
            n3084 = local read "S 39"() -> (w4010:string)
            n3085 = local read "S 38"() -> (w4017:string)
            n3086 = local read "Temperature before test 2"() -> (w4048:dbl)
            n3087 = local read "Temperature after test 2"() -> (w4038:dbl)
            n3088 = local read "Humidity before test 2"() -> (w4063:dbl)
            n3089 = local read "Humidity after test 2"() -> (w4047:dbl)
            n3090 = local read "MWSD 2"() -> (w4052:dbl)
            n3091 = local read "WS1.4 2"() -> (w4030:dbl)
            n3092 = Concatenate Strings("2)" ("string"), w4012) -> (w4013:string)
            n3093 = Concatenate Strings("3)" ("string"), w4010) -> (w4011:string)
            n3094 = Concatenate Strings("1)" ("string"), w4017) -> (w4016:string)
            n3095 = Concatenate Strings("4)" ("string"), w4007) -> (w4008:string)
            n3096 = Concatenate Strings("5)" ("string"), w4005) -> (w4004:string)
            n3097 = Concatenate Strings("6)" ("string"), w4002) -> (w4001:string)
            n3098 = Concatenate Strings("7)" ("string"), w3998) -> (w3999:string)
            n3099 = Concatenate Strings("8)" ("string"), w3995) -> (w3996:string)
            n3100 = local read "HCF 2"() -> (w4034:dbl)
            n3101 = local read "AVP 2"() -> (w4051:dbl)
            n3102 = local read "s.NO"() -> (w3993:string)
            n3103 = call <vilib>:"New Report.vi"("report type"=enum16{"Standard Report", "HTML"}."Standard Report") -> ("report out"=w4072:refnum<class "NI_report.lvclass">, "error out"=w4071:errorcluster)  [unwired: 13 in]
            n3104 = local read "TITTLE"() -> (w4024:string)
            n3105 = Concatenate Strings(w4049, w3992, w3993, w4049, w4027, w4022, w4049, w4026, w4023, w4049, w4028, w4025, w4049) -> (w4042:string)
            "test by" <- w4042
            n3106 = Number To Fractional String(number=w4048, width (-)=i16 6, precision (6)=i16 2) -> (F-format string=w4037:string)  [unwired: 1 in]
            n3107 = Number To Fractional String(number=w4047, width (-)=i16 6, precision (6)=i16 2) -> (F-format string=w4050:string)  [unwired: 1 in]
            n3108 = Number To Fractional String(number=w4063, width (-)=i16 6, precision (6)=i16 2) -> (F-format string=w4068:string)  [unwired: 1 in]
            n3109 = Number To Fractional String(number=w4052, width (-)=i16 6, precision (6)=i16 2) -> (F-format string=w4054:string)  [unwired: 1 in]
            n3110 = Number To Fractional String(number=w4038, width (-)=i16 6, precision (6)=i16 2) -> (F-format string=w4039:string)  [unwired: 1 in]
            n3111 = Number To Fractional String(number=w4051, width (-)=i16 6, precision (6)=i16 2) -> (F-format string=w4053:string)  [unwired: 1 in]
            n3112 = Number To Fractional String(number=w4034, width (-)=i16 6, precision (6)=i16 2) -> (F-format string=w4033:string)  [unwired: 1 in]
            n3113 = Number To Fractional String(number=w4030, precision (6)=i16 2) -> (F-format string=w4029:string)  [unwired: 2 in]
            n3114 = call-dynamic "Set Report Header Text.vi"("report in"=w4072, "center header text"=w4024, "error in (no error)"=w4071) -> ("report out"=w4043:refnum<class "NI_report.lvclass">, "error out"=w4044:errorcluster)  [unwired: 11 in]
            n3115 = Concatenate Strings(w4032, w4016, w4068, w4032, w4013, w4037, w4032, w4011, w4050, w4032, w4008, w4039, w4032, w4004, w4054, w4032, w4001, w4053, w4032, w3999, w4033, w4032, w3996, w4029) -> (w4020:string)
            "export 2" <- w4020
            n3116 = call-poly <vilib>:"Append Report Text.vi"("report in"=w4043, "text"=w4042, "error in (no error)"=w4044) -> ("report out"=w4046:refnum<class "NI_report.lvclass">, "error out"=w4045:errorcluster)  [unwired: 9 in, 2 out]
            n3117 = local read "test by"() -> (w4019:string)
            n3118 = local read "TITTLE"() -> (w4021:string)
            n3119 = call-poly <vilib>:"Append Report Text.vi"("report in"=w4046, "error in (no error)"=w4045) -> ("report out"=w4067:refnum<class "NI_report.lvclass">, "error out"=w4065:errorcluster)  [unwired: 10 in, 2 out]
            n3120 = Concatenate Strings(w4021, w4020, w4019) -> (→"output":string)
            n3121 = call-poly <vilib>:"Append Report Text.vi"("report in"=w4067, "text"=w4020, "error in (no error)"=w4065) -> ("report out"=w4066:refnum<class "NI_report.lvclass">, "error out"=w4064:errorcluster)  [unwired: 9 in, 2 out]
            n3122 = call-dynamic "Print Report.vi"("report in"=w4066, "printer name (default)"=w4074, "error in (no error)"=w4064) -> ("report out"=w4076:refnum<class "NI_report.lvclass">, "error out"=w4077:errorcluster)  [unwired: 11 in]
            n3123 = call-dynamic "Dispose Report.vi"("report in"=w4076, "error in (no error)"=w4077) -> ()  [unwired: 13 in, 1 out]
          }
        }
        n3124 = case shown="True" "Print 2" {
          frame False {
          }
          frame True {
            n3125 = flat-sequence {
              frame #0 {
                n3126 = local read "s.NO"() -> (→"s.NO 2":string)
                n3127 = Wait (ms)(milliseconds to wait=u32 20) -> ()  [unwired: 1 out]
                n3128 = local read "Sample ID  3"() -> (→"Sample ID  6":string)
                n3129 = local read "Sample ID  4"() -> (→"Sample ID  7":string)
                n3130 = local read "Sample ID"() -> (→"Sample ID  2":string)
                n3131 = local read "Tested by"() -> (→"Tested by 2":string)
                n3132 = local read "Test Date"() -> (→"Test Date 2":string)
                n3133 = local read "Humidity after test 3"() -> (→"Humidity after test 4":dbl)
                n3134 = local read "Ref A Test Date :"() -> (→"TITTLE 4":string)
                n3135 = local read "Temperature before test 3"() -> (w3899:dbl)
                n3136 = local read "Temperature before test 3"() -> (→"Temperature after test 5":dbl)
                n3137 = local read "Temperature after test 3"() -> (→"Temperature after test 4":dbl)
                n3138 = local read "Humidity before test 3"() -> (→"Humidity before test 4":dbl)
                n3139 = local write "Temperature before test 3"(w3899) -> ()
                n3140 = local read "image data"() -> (w3890:T16)
                n3141 = String To Path(string="C:\\LAB-IQ\\im\\Temp_resized.jpg") -> (path=w3891:path)
                "path 2" <- w3891
                n3142 = call <vilib>:"Write JPEG File.vi"("image data"=w3890, "path to JPEG file"=w3891) -> ()  [unwired: 8 in, 2 out]
                "Ref A Test Date :" <- "Ref A Test Date :"
                "Ref B Test Date :" <- "Ref B Test Date :"
                "Ref B Scar Value :" <- "Ref B Scar Value :"
                "Ref A Scar Value :" <- "Ref A Scar Value :"
              }
              frame #1 {
                (unwired) HTML_Report_Image_Alignment."MIDDLE" ("alignment (default)")
                w3927 = u16 0 items=["portrait", "landscape"] ("orientation (portrait)")
                (unwired) HTML_Report_Image_Alignment."ABSMIDDLE" ("alignment (default)")
                (unwired) "TESTED BY : "
                (unwired) "TESTED DATE :"
                (unwired) "SAMPLE ID : "
                (unwired) "SAMPLE DESIGN : "
                w3960 = "\r"
                # "add image"
                n3143 = Wait (ms)(milliseconds to wait=u32 20) -> ()  [unwired: 1 out]
                n3144 = local read "Sample ID  2"() -> (w3953:string)
                n3145 = local read "Wear Scar X"() -> (w3925:dbl)
                "Length ( microns ) 2" <- w3925
                n3146 = local read "Wear Scar Y"() -> (w3924:dbl)
                "Wear Scar Y ( microns ) :" <- w3924
                n3147 = local read "Test Date 2"() -> (w3954:string)
                n3148 = local read "Tested by 2"() -> (w3955:string)
                n3149 = local read "String 46"() -> (w3951:string)
                n3150 = local read "String 48"() -> (w3957:string)
                n3151 = local read "String 47"() -> (w3956:string)
                n3152 = local read "String 49"() -> (w3958:string)
                n3153 = local read "String 10"() -> (w3911:string)
                n3154 = local read "s.NO 2"() -> (w3952:string)
                n3155 = Add(x=w3925, y=w3924) -> (x+y=w3923:dbl)
                n3156 = call <vilib>:"New Report.vi"("report type"=enum16{"Standard Report", "HTML"}."HTML") -> ("report out"=w3931:refnum<class "NI_report.lvclass">, "error out"=w3929:errorcluster)  [unwired: 13 in]
                n3157 = Concatenate Strings(w3960, w3951, w3952, w3960, w3957, w3953, w3960, w3956, w3954, w3960, w3958, w3955, w3960) -> (→"test by 2":string)
                n3158 = Concatenate Strings("C:\\LAB-IQ\\Data\\" ("string"), w3911, ".jpg" ("string")) -> ()  [unwired: 1 out]
                n3159 = Divide(x=w3923, y=2.0) -> (x/y=→"Mean Wear ( microns) :":dbl)
                n3160 = call-dynamic "Set Report Orientation.vi"("report in"=w3931, "orientation (portrait)"=w3927, "error in (no error)"=w3929) -> ("report out"=w3930:refnum<class "NI_report.lvclass">, "error out"=w3928:errorcluster)  [unwired: 11 in]
                n3161 = for {
                  N: 5 -> [_]
                  tunnel: w3930 -> [w3981]
                  tunnel: [w3980] -> w3909
                  tunnel: w3928 -> [w3979]
                  tunnel: [w3978] -> w3908
                  n3162 = call-dynamic "Set Report Tab Width.vi"("report in"=w3981, "error in (no error)"=w3979) -> ("report out"=w3980:refnum<class "NI_report.lvclass">, "error out"=w3978:errorcluster)  [unwired: 12 in]
                }